vi "UHR-Fleezers Control (host) - 12.7.vi"() -> ()   [LabVIEW 2012] (continued)
        n2479 = To Double Precision Float(number=w3747) -> (double precision float=w3746:dbl[])
        n2480 = To Double Precision Float(number=w3745) -> (double precision float=w3744:dbl[])
        n2481 = Index Array(array=w3872, index=10) -> (element=w3878:waveform(dbl))
        n2482 = Index Array(array=w3872, index=11) -> (element=w3875:waveform(dbl))
        n2483 = local read "Cycles/step (MCL)"() -> (w3828:u64)
        n2484 = Index Array(array=w3872, index="Channel") -> (element=w3874:waveform(dbl))
        n2485 = Unbundle(w3780) -> ("New Image"=w3779:T2, "New Image"=w3778:T2, "New Image"=w3751:T2, "New Image"=w3752:T2, "New Image"=w3753:T2)
        n2486 = local read "Scan steps (MCL)"() -> (w3739:u64)
        n2487 = Unbundle By Name(w3878) -> ("Y"=w3830:dbl[])
        n2488 = Unbundle By Name(w3875) -> ("Y"=w3832:dbl[])
        n2489 = local read "Scan lines (y)"() -> (w3740:u64)
        n2490 = local read "N APD Samp/step"() -> (w3742:dbl)
        n2491 = Unbundle By Name(w3874) -> ("Y"=w3837:dbl[])
        n2492 = call "downsample 1D array - double.vi"("Ave N"=w3828, "Array In"=w3830) -> ("Array Out"=w3829:dbl[])  [unwired: 1 out]
        n2493 = call "downsample 1D array - double.vi"("Ave N"=w3828, "Array In"=w3832) -> ("Array Out"=w3831:dbl[])  [unwired: 1 out]
        n2494 = call "downsample 1D array - double.vi"("Ave N"=w3828, "Array In"=w3837) -> ("Array Out"=w3836:dbl[])  [unwired: 1 out]
        n2495 = Multiply(x=w3739, y=u64 2) -> (x*y=w3741:u64)
        n2496 = feedback #11(w3746) -> (w3805:dbl[])
        n2497 = Build Array (concatenate)(w3805, w3746) -> (w3804:dbl[])
        n2498 = feedback #12(w3744) -> (w3777:dbl[])
        n2499 = Build Array (concatenate)(w3777, w3744) -> (w3738:dbl[])
        n2500 = Select(t=w3746, s=w3743, f=w3804) -> (s? t:f=w3789:dbl[])
        n2501 = feedback-in #11(w3789) -> ()
        n2502 = Select(t=w3744, s=w3743, f=w3738) -> (s? t:f=w3762:dbl[])
        n2503 = feedback-in #12(w3762) -> ()
        n2504 = feedback #13(w3748) -> (w3898:dbl[])
        n2505 = Build Array (concatenate)(w3898, w3748) -> (w3880:dbl[])
        n2506 = Select(t=w3748, s=w3743, f=w3880) -> (s? t:f=w3884:dbl[])
        n2507 = feedback-in #13(w3884) -> ()
        n2508 = feedback #14(w3829) -> (w3886:dbl[])
        n2509 = Build Array (concatenate)(w3886, w3829) -> (w3877:dbl[])
        n2510 = feedback #15(w3836) -> (w3896:dbl[])
        n2511 = Build Array (concatenate)(w3896, w3836) -> (w3895:dbl[])
        n2512 = feedback #16(w3831) -> (w3888:dbl[])
        n2513 = Build Array (concatenate)(w3888, w3831) -> (w3889:dbl[])
        n2514 = Select(t=w3829, s=w3743, f=w3877) -> (s? t:f=w3833:dbl[])
        n2515 = feedback-in #14(w3833) -> ()
        n2516 = Select(t=w3836, s=w3743, f=w3895) -> (s? t:f=w3835:dbl[])
        n2517 = feedback-in #15(w3835) -> ()
        n2518 = Select(t=w3831, s=w3743, f=w3889) -> (s? t:f=w3834:dbl[])
        n2519 = feedback-in #16(w3834) -> ()
        n2520 = call "integrate 1D array interval - double.vi"("Ave N"=w3742, "Array In"=w3789) -> ("Array Out"=w3800:dbl[])  [unwired: 1 out]
        n2521 = call "integrate 1D array interval - double.vi"("Ave N"=w3742, "Array In"=w3762) -> ("Array Out"=w3773:dbl[])  [unwired: 1 out]
        n2522 = call "integrate 1D array interval - double.vi"("Ave N"=w3742, "Array In"=w3884) -> ("Array Out"=w3883:dbl[])  [unwired: 1 out]
        n2523 = Array Size(array=w3800) -> (size(s)=w3801:i32)
        n2524 = Array Size(array=w3773) -> (size(s)=w3774:i32)
        n2525 = Array Size(array=w3883) -> (size(s)=w3885:i32)
        n2526 = Multiply(x=w3740, y=w3741) -> (x*y=w3803:u64)
        n2527 = Multiply(x=w3740, y=w3741) -> (x*y=w3776:u64)
        n2528 = Multiply(x=w3740, y=w3741) -> (x*y=w3893:u64)
        n2529 = Subtract(x=w3803, y=w3801) -> (x-y=w3794:u64)
        n2530 = call-poly <vilib>:"Mean.vi"("X"=w3800) -> ("mean"=w3791:dbl)  [unwired: 1 out]
        n2531 = Subtract(x=w3776, y=w3774) -> (x-y=w3767:u64)
        n2532 = call-poly <vilib>:"Mean.vi"("X"=w3773) -> ("mean"=w3764:dbl)  [unwired: 1 out]
        n2533 = Subtract(x=w3893, y=w3885) -> (x-y=w3827:u64)
        n2534 = call-poly <vilib>:"Mean.vi"("X"=w3883) -> ("mean"=w3824:dbl)  [unwired: 1 out]
        n2535 = call-poly <vilib>:"Mean.vi"("X"=w3833) -> ("mean"=w3817:dbl)  [unwired: 1 out]
        n2536 = call-poly <vilib>:"Mean.vi"("X"=w3835) -> ("mean"=w3822:dbl)  [unwired: 1 out]
        n2537 = call-poly <vilib>:"Mean.vi"("X"=w3834) -> ("mean"=w3820:dbl)  [unwired: 1 out]
        n2538 = Initialize Array(1.0 ("element"), w3794) -> (w3790:dbl[])
        n2539 = Initialize Array(1.0 ("element"), w3767) -> (w3763:dbl[])
        n2540 = Initialize Array(1.0 ("element"), w3827) -> (w3818:dbl[])
        n2541 = Multiply(x=w3790, y=w3791) -> (x*y=w3792:dbl[])
        n2542 = Multiply(x=w3763, y=w3764) -> (x*y=w3765:dbl[])
        n2543 = Multiply(x=w3818, y=w3824) -> (x*y=w3825:dbl[])
        n2544 = Multiply(x=w3818, y=w3820) -> (x*y=w3821:dbl[])
        n2545 = Multiply(x=w3818, y=w3822) -> (x*y=w3823:dbl[])
        n2546 = Multiply(x=w3818, y=w3817) -> (x*y=w3819:dbl[])
        n2547 = Build Array (concatenate)(w3800, w3792) -> (w3802:dbl[])
        n2548 = Build Array (concatenate)(w3773, w3765) -> (w3775:dbl[])
        n2549 = Build Array (concatenate)(w3883, w3825) -> (w3892:dbl[])
        n2550 = Build Array (concatenate)(w3833, w3819) -> (w3887:dbl[])
        n2551 = Build Array (concatenate)(w3835, w3823) -> (w3891:dbl[])
        n2552 = Build Array (concatenate)(w3834, w3821) -> (w3890:dbl[])
        n2553 = Reshape Array(w3802, w3740, w3741) -> (w3798:dbl[][])
        n2554 = Reshape Array(w3775, w3740, w3741) -> (w3771:dbl[][])
        n2555 = Reshape Array(w3892, w3740, w3741) -> (w3870:dbl[][])
        n2556 = Reshape Array(w3887, w3740, w3741) -> (w3853:dbl[][])
        n2557 = Reshape Array(w3891, w3740, w3741) -> (w3845:dbl[][])
        n2558 = Reshape Array(w3890, w3740, w3741) -> (w3860:dbl[][])
        n2559 = Array Subset(array=w3798, index (col)=0 ("index"), length (col)=w3739) -> (w3797:dbl[][])  [unwired: 2 in]
        n2560 = Array Subset(array=w3798, index (col)=w3739) -> (w3795:dbl[][])  [unwired: 3 in]
        n2561 = Array Subset(array=w3771, index (col)=0 ("index"), length (col)=w3739) -> (w3770:dbl[][])  [unwired: 2 in]
        n2562 = Array Subset(array=w3771, index (col)=w3739) -> (w3768:dbl[][])  [unwired: 3 in]
        n2563 = Array Subset(array=w3860, index (col)=0 ("index"), length (col)=w3739) -> (w3865:dbl[][])  [unwired: 2 in]
        n2564 = Array Subset(array=w3860, index (col)=w3739) -> (w3863:dbl[][])  [unwired: 3 in]
        n2565 = Array Subset(array=w3870, index (col)=0 ("index"), length (col)=w3739) -> (w3869:dbl[][])  [unwired: 2 in]
        n2566 = Array Subset(array=w3870, index (col)=w3739) -> (w3867:dbl[][])  [unwired: 3 in]
        n2567 = Array Subset(array=w3845, index (col)=0 ("index"), length (col)=w3739) -> (w3851:dbl[][])  [unwired: 2 in]
        n2568 = Array Subset(array=w3845, index (col)=w3739) -> (w3849:dbl[][])  [unwired: 3 in]
        n2569 = Array Subset(array=w3853, index (col)=0 ("index"), length (col)=w3739) -> (w3858:dbl[][])  [unwired: 2 in]
        n2570 = Array Subset(array=w3853, index (col)=w3739) -> (w3856:dbl[][])  [unwired: 3 in]
        n2571 = for {
          tunnel: w3797 -> [w3902] mode=indexing
          tunnel: [w3901] -> w3796 mode=indexing
          workers-P: _ -> [_]
          n2572 = Reverse 1D Array(array=w3902) -> (reversed array=w3901:dbl[])
        }
        n2573 = for {
          tunnel: w3770 -> [w3900] mode=indexing
          tunnel: [w3899] -> w3769 mode=indexing
          workers-P: _ -> [_]
          n2574 = Reverse 1D Array(array=w3900) -> (reversed array=w3899:dbl[])
        }
        n2575 = for {
          tunnel: w3865 -> [w3908] mode=indexing
          tunnel: [w3907] -> w3864 mode=indexing
          workers-P: _ -> [_]
          n2576 = Reverse 1D Array(array=w3908) -> (reversed array=w3907:dbl[])
        }
        n2577 = for {
          tunnel: w3869 -> [w3910] mode=indexing
          tunnel: [w3909] -> w3868 mode=indexing
          workers-P: _ -> [_]
          n2578 = Reverse 1D Array(array=w3910) -> (reversed array=w3909:dbl[])
        }
        n2579 = for {
          tunnel: w3851 -> [w3904] mode=indexing
          tunnel: [w3903] -> w3850 mode=indexing
          workers-P: _ -> [_]
          n2580 = Reverse 1D Array(array=w3904) -> (reversed array=w3903:dbl[])
        }
        n2581 = for {
          tunnel: w3858 -> [w3906] mode=indexing
          tunnel: [w3905] -> w3857 mode=indexing
          workers-P: _ -> [_]
          n2582 = Reverse 1D Array(array=w3906) -> (reversed array=w3905:dbl[])
        }
        n2583 = Index Array(array=w3870, index (row)=0) -> (element=→"Waveform Graph":dbl[])  [unwired: 1 in]
        n2584 = Add(x=w3796, y=w3795) -> (x+y=w3782:dbl[][])
        n2585 = Add(x=w3769, y=w3768) -> (x+y=w3755:dbl[][])
        n2586 = Add(x=w3864, y=w3863) -> (x+y=w3862:dbl[][])
        n2587 = Add(x=w3868, y=w3867) -> (x+y=w3842:dbl[][])
        n2588 = Add(x=w3850, y=w3849) -> (x+y=w3848:dbl[][])
        n2589 = Add(x=w3857, y=w3856) -> (x+y=w3855:dbl[][])
        n2590 = Divide(x=w3848, y=2) -> (x/y=w3846:dbl[][])
        n2591 = Divide(x=w3862, y=2) -> (x/y=w3807:dbl[][])
        n2592 = To Single Precision Float(number=w3842) -> (single precision float=w3841:sgl[][])
        n2593 = To Single Precision Float(number=w3782) -> (single precision float=w3786:sgl[][])
        n2594 = To Single Precision Float(number=w3755) -> (single precision float=w3759:sgl[][])
        n2595 = Divide(x=w3855, y=2) -> (x/y=w3809:dbl[][])
        n2596 = Transpose 2D Array(2D array=w3846) -> (transposed array=→"Data map":dbl[][])
        n2597 = To Single Precision Float(number=w3807) -> (single precision float=w3813:sgl[][])
        n2598 = To Single Precision Float(number=w3809) -> (single precision float=w3810:sgl[][])
        n2599 = call "IMAQ ArrayToImage"("Image Pixels (Float)"=w3841, "Image"=w3779) -> ("Image Out"=w3844:T2)  [unwired: 8 in, 1 out]
        n2600 = call "IMAQ ArrayToImage"("Image Pixels (Float)"=w3786, "Image"=w3778) -> ("Image Out"=w3788:T2)  [unwired: 8 in, 1 out]
        n2601 = call "IMAQ ArrayToImage"("Image Pixels (Float)"=w3759, "Image"=w3751) -> ("Image Out"=w3761:T2)  [unwired: 8 in, 1 out]
        n2602 = call "IMAQ ArrayToImage"("Image Pixels (Float)"=w3813, "Image"=w3752) -> ("Image Out"=w3815:T2)  [unwired: 8 in, 1 out]
        n2603 = call "IMAQ Symmetry"("Type of Symmetry"=w3843, "Image Src"=w3844) -> ("Image Dst Out"=w3839:T2)  [unwired: 3 in, 1 out]
        n2604 = call "IMAQ ArrayToImage"("Image Pixels (Float)"=w3810, "Image"=w3753) -> ("Image Out"=w3812:T2)  [unwired: 8 in, 1 out]
        n2605 = call "IMAQ Symmetry"("Type of Symmetry"=w3787, "Image Src"=w3788) -> ("Image Dst Out"=w3784:T2)  [unwired: 3 in, 1 out]
        n2606 = call "IMAQ Symmetry"("Type of Symmetry"=w3760, "Image Src"=w3761) -> ("Image Dst Out"=w3757:T2)  [unwired: 3 in, 1 out]
        n2607 = call "IMAQ Symmetry"("Type of Symmetry"=w3814, "Image Src"=w3815) -> ("Image Dst Out"=→"Detection Laser X":T2)  [unwired: 3 in, 1 out]
        n2608 = call "IMAQ Symmetry"("Type of Symmetry"=w3811, "Image Src"=w3812) -> ("Image Dst Out"=→"Detection Laser Y":T2)  [unwired: 3 in, 1 out]
        n2609 = call "IMAQ Set Simple Calibration"("Calibration Axis Info"=T36 {"Origin Pixel"={"X"=0.0, "Y"=0.0}, "Angle Relative to Horizontal (deg)"=0.0, "Axis Reference"=0}, "Grid Descriptor"=T37 {"X Step"=0.3, "Y Step"=0.3, "Unit"=enum."Undefined"}, "Image"=w3839) -> ("Calibrated Image"=→"APD 1":T2)  [unwired: 7 in, 1 out]
        n2610 = call "IMAQ Set Simple Calibration"("Calibration Axis Info"=T36 {"Origin Pixel"={"X"=0.0, "Y"=0.0}, "Angle Relative to Horizontal (deg)"=0.0, "Axis Reference"=0}, "Grid Descriptor"=T37 {"X Step"=0.3, "Y Step"=0.3, "Unit"=enum."Undefined"}, "Image"=w3784) -> ("Calibrated Image"=→"APD 2":T2)  [unwired: 7 in, 1 out]
        n2611 = call "IMAQ Set Simple Calibration"("Calibration Axis Info"=T36 {"Origin Pixel"={"X"=0.0, "Y"=0.0}, "Angle Relative to Horizontal (deg)"=0.0, "Axis Reference"=0}, "Grid Descriptor"=T37 {"X Step"=0.3, "Y Step"=0.3, "Unit"=enum."Undefined"}, "Image"=w3757) -> ("Calibrated Image"=→"APD 3":T2)  [unwired: 7 in, 1 out]
      }
    }
    n2612 = case "For computing FFTs for display" shown="True" "Compute FFT" {
      tunnel: w3256 -> [_ w4382]
      frame False {
      }
      frame True {
        n2613 = Build Array("FFT 1 Choice 1", "FFT 1 Choice 2", "FFT 2 Choice 1", "FFT 2 Choice 2") -> (w4375:u16[])
        n2614 = Array Size(array=w4382) -> (size(s)=w4381:i32)
        n2615 = feedback-in #17(w4375) -> ()
        n2616 = feedback #17(u16[] [100, 100, 100, 100]) -> (w4376:u16[])
        n2617 = feedback-in #18("# Spectra to Ave.") -> ()
        n2618 = feedback #18("# Spectra to Ave.") -> (w4373:dbl)
        n2619 = Not Equal?(x="# Spectra to Ave.", y=w4373) -> (x != y?=w4372:bool)
        n2620 = Not Equal?(x=w4375, y=w4376) -> (x != y?=w4374:bool)
        n2621 = feedback #19(1.0) -> (w4359:dbl)
        n2622 = Compound Arithmetic op=OR("Reset FFT", w4374, w4372) -> (w4357:bool)
        n2623 = Select(t=1.0, s=w4357, f=w4359) -> (s? t:f=w4361:dbl)
        n2624 = Greater?(x=w4361, y="# Spectra to Ave.") -> (0:w4380:bool)
        n2625 = Increment(x=w4361) -> (x+1=w4360:dbl)
        n2626 = feedback-in #19(w4360) -> ()
        n2627 = local read "DMA Update Period (s)"() -> (w4355:dbl)
        n2628 = Multiply(x="# Spectra to Ave.", y=w4355) -> (x*y=→"Ave. Time (s)":dbl)
        n2629 = Build Array(cluster{"f0":dbl, "df":dbl, "magnitude":dbl[]} {"f0"=0.0, "df"=0.0, "magnitude"=[]} ("PSD")) -> (w4364:cluster{"f0":dbl, "df":dbl, "magnitude":dbl[]}[])
        n2630 = Build Array(w4364, w4364, w4364, w4364) -> (w4366:T46)
        n2631 = feedback #20(w4366) -> (w4371:T46)
        n2632 = for {
          N: 4 -> [_]
          tunnel: w4375 -> [w4404] mode=indexing
          tunnel: w4382 -> [w4405]
          tunnel: w4381 -> [w4407]
          tunnel: w4357 -> [w4400]
          tunnel: w4380 -> [w4399]
          tunnel: "# Spectra to Ave." -> [w4398]
          tunnel: [w4397] -> w4370 mode=indexing
          tunnel: w4371 -> [w4402] mode=indexing
          tunnel: [w4401] -> w4358 mode=indexing
          tunnel: w4361 -> [w4396]
          n2633 = Less?(x=w4404, y=w4407) -> (x < y?=w4406:bool)
          n2634 = Index Array(array=w4405, index=w4404) -> (element=w4403:waveform(dbl))
          n2635 = case shown="True" w4406 {
            tunnel: w4403 -> [_ w4424]
            tunnel: w4402 -> [w4409 w4422]
            tunnel: [w4409 w4410] -> w4401
            tunnel: w4400 -> [_ w4421]
            tunnel: w4399 -> [_ w4414]
            tunnel: w4398 -> [_ w4413]
            tunnel: [cluster{"f0":dbl, "df":dbl, "magnitude":dbl[]} {"f0"=0.0, "df"=0.0, "magnitude"=[]} ("PSD") w4415] -> w4397
            tunnel: w4396 -> [_ w4412]
            frame False {
            }
            frame True {
              n2636 = call <vilib>:"Std Deviation and Variance.vi"("X"=w4424) -> ("mean"=w4425:dbl)  [unwired: 1 in, 2 out]
              n2637 = Subtract(x=w4424, y=w4425) -> (x-y=w4423:waveform(dbl))
              n2638 = xnode "Spectral Measurements"("Signals"=w4423) -> ("PSD"=w4417:cluster{"f0":dbl, "df":dbl, "magnitude":dbl[]})  [unwired: 1 in, 1 out]
              n2639 = case shown="False" w4421 {
                tunnel: w4422 -> [w4434 _]
                tunnel: [w4430 w4439] -> w4410
                tunnel: w4417 -> [w4433 w4440]
                tunnel: w4414 -> [w4432 _]
                frame False {
                  n2640 = Build Array (concatenate)(w4434, w4433) -> (w4431:cluster{"f0":dbl, "df":dbl, "magnitude":dbl[]}[])
                  n2641 = case shown="True" w4432 {
                    tunnel: w4431 -> [w4435 w4438]
                    tunnel: [w4435 w4436] -> w4430
                    frame False {
                    }
                    frame True {
                      n2642 = Delete From Array(array=w4438, index=0) -> (array with subset deleted=w4436:cluster{"f0":dbl, "df":dbl, "magnitude":dbl[]}[])  [unwired: 1 in, 1 out]
                    }
                  }
                }
                frame True {
                  n2643 = Build Array(w4440) -> (w4439:cluster{"f0":dbl, "df":dbl, "magnitude":dbl[]}[])
                }
              }
              n2644 = for {
                tunnel: w4410 -> [w4429] mode=indexing
                tunnel: [w4428] -> w4420 mode=indexing
                workers-P: _ -> [_]
                n2645 = Unbundle By Name(w4429) -> ("magnitude"=w4428:dbl[])
              }
              n2646 = Transpose 2D Array(2D array=w4420) -> (transposed array=w4419:dbl[][])
              n2647 = for {
                tunnel: w4419 -> [w4427] mode=indexing
                tunnel: [w4426] -> w4418 mode=indexing
                workers-P: _ -> [_]
                n2648 = Add Array Elements(numeric array=w4427) -> (sum=w4426:dbl)
              }
              n2649 = Select(t=w4413, s=w4414, f=w4412) -> (s? t:f=w4411:dbl)
              n2650 = Divide(x=w4418, y=w4411) -> (x/y=w4416:dbl[])
              n2651 = Bundle By Name(cluster=w4417, "magnitude"=w4416) -> (w4415:cluster{"f0":dbl, "df":dbl, "magnitude":dbl[]})
            }
          }
        }
        n2652 = case shown="True" w4357 {
          tunnel: w4358 -> [w4389 w4395]
          tunnel: [w4389 w4390] -> w4356
          frame False {
          }
          frame True {
            n2653 = Array Subset(array=w4395, index (row)=0 ("index"), length (row)=4 ("length"), index (col)=0 ("index"), length (col)=1 ("length")) -> (w4390:T46)
          }
        }
        n2654 = feedback-in #20(w4356) -> ()
        n2655 = Split 1D Array(array=w4370, index=2) -> (first subarray=→"FFT 1":cluster{"f0":dbl, "df":dbl, "magnitude":dbl[]}[], second subarray=→"FFT 2":cluster{"f0":dbl, "df":dbl, "magnitude":dbl[]}[])
      }
    }
    n2656 = Index Array(array=w3254, index=4) -> (element=w3310:waveform(dbl))
    n2657 = Index Array(array=w3254, index=7) -> (element=w3307:waveform(dbl))
    n2658 = Divide(x="T1 offset_x (mV)", y=1000.0) -> (x/y=w3311:dbl)
    n2659 = feedback-in #21("Calibration") -> ()
    n2660 = feedback #21(u16 1 ("Calibration")) -> (w3329:u16)
    n2661 = Divide(x="T2 offset_x (mV)", y=1000.0) -> (x/y=w3309:dbl)
    n2662 = case shown="2" "Calibration" {
      tunnel: "T1 alpha_x (nm/V)" -> [_ w3703 w3724]
      tunnel: "T1 kappa_x (pN/nm)" -> [_ _ w3714]
      tunnel: "T2 alpha_x (nm/V)" -> [_ w3702 w3722]
      tunnel: "T2 kappa_x (pN/nm)" -> [_ _ w3715]
      tunnel: w3310 -> [w3685 w3700 w3720]
      tunnel: w3307 -> [w3684 w3698 w3718]
      tunnel: [w3685 w3697 w3717] -> w3338
      tunnel: [w3684 w3696 w3716] -> w3337
      tunnel: ["T1 X (V)" ("Label.Text") "T1 X (nm)" ("Label.Text") "T1 X (pN)" ("Label.Text")] -> w3326
      tunnel: ["T2 X (V)" ("Label.Text") "T2 X (nm)" ("Label.Text") "T2 X (pN)" ("Label.Text")] -> w3325
      tunnel: ["Position (V)" ("Label.Text") "Position (nm)" ("Label.Text") "Force (pN)" ("Label.Text")] -> w3327
      tunnel: w3309 -> [_ w3688 w3707]
      tunnel: w3311 -> [_ w3691 w3709]
      tunnel: ["Mean (V)" ("Label.Text") "Mean (nm)" ("Label.Text") "Mean (pN)" ("Label.Text")] -> w3322
      tunnel: ["Difference (V)" ("Label.Text") "Difference (nm)" ("Label.Text") "Difference (pN)" ("Label.Text")] -> w3262
      frame 0, Default {
      }
      frame 1 {
        n2663 = Unbundle By Name(w3700) -> ("Y"=w3704:dbl[])
        n2664 = Unbundle By Name(w3698) -> ("Y"=w3689:dbl[])
        n2665 = Subtract(x=w3704, y=w3691) -> (x-y=w3692:dbl[])
        n2666 = Subtract(x=w3689, y=w3688) -> (x-y=w3690:dbl[])
        n2667 = Multiply(x=w3690, y=w3702) -> (x*y=w3699:dbl[])
        n2668 = Multiply(x=w3703, y=w3692) -> (x*y=w3701:dbl[])
        n2669 = Bundle By Name(cluster=w3698, "Y"=w3699) -> (w3696:waveform(dbl))
        n2670 = Bundle By Name(cluster=w3700, "Y"=w3701) -> (w3697:waveform(dbl))
      }
      frame 2 {
        n2671 = Unbundle By Name(w3720) -> ("Y"=w3725:dbl[])
        n2672 = Unbundle By Name(w3718) -> ("Y"=w3723:dbl[])
        n2673 = Subtract(x=w3723, y=w3707) -> (x-y=w3708:dbl[])
        n2674 = Subtract(x=w3725, y=w3709) -> (x-y=w3710:dbl[])
        n2675 = Compound Arithmetic op=MULTIPLY(w3708, w3722, w3715) -> (w3719:dbl[])
        n2676 = Compound Arithmetic op=MULTIPLY(w3714, w3724, w3710) -> (w3721:dbl[])
        n2677 = Bundle By Name(cluster=w3718, "Y"=w3719) -> (w3716:waveform(dbl))
        n2678 = Bundle By Name(cluster=w3720, "Y"=w3721) -> (w3717:waveform(dbl))
      }
    }
    n2679 = case shown="True" "Read Lateness and Rel Phase" {
      tunnel: w3128 -> [w3640 w3673]
      tunnel: w3127 -> [w3641 w3672]
      tunnel: [w3640 w3645] -> w3304
      tunnel: [w3641 w3644] -> w3303
      frame False {
      }
      frame True {
        n2680 = xnode "Read/Write Control"("FPGA VI Reference In"=w3673, "error in"=w3672) -> ("FPGA VI Reference Out"=w3647:T20, "error out"=w3646:errorcluster, "GI Relative phase"=→"GI relative phase":i16, "Relative phase"=→"Relative phase (AI1)":i16, "AI Late Counter"=→"Late Counter (AI1)":u8, "GI Late Counter"=→"GI Late Counter":u8, "MCL Late Counter"=→"MCL Late Counter":u8, "MCL Relative Phase"=→"Relative Phase (MCL)":i16, "APD Acq Relative Phase"=→"APD Acq Relative Phase":i16, "APD 1 Gate Relative Phase"=→"APD 1 Gate Relative Phase":i16, "APD 2 Gate Relative Phase"=→"APD 2 Gate Relative Phase":i16, "APD Acq Late Counter"=→"APD Acq Late Counter":u8, "APD 1 Gate Late Counter"=→"APD 1 Gate Late Counter":u8, "APD 2 Gate Late Counter"=→"APD 2 Gate Late Counter":u8, "Green FB Relative Phase"=→"Relative phase (Green FB)":i16, "GI Relative phase 2"=→"GI relative phase 2":i16, "GI Late Counter 2"=→"GI Late Counter 2":u8, "Trap Pos FIFO Timeout"=→"Trap Pos FIFO Timeout":u16, "Trap AI FIFO Timeout"=→"Trap AI FIFO Timeout":u16, "RI Late Counter"=→"RI Late Counter":u8, "RI Relative phase"=→"RI relative phase":i16, "Green Late Counter"=→"Green AI Late Counter":u8, "BI Late Counter (AO)"=→"Late Counter (BI AO)":u8, "Blue Late Counter (D)"=→"Late Counter (BI DO)":u8, "BI Relative phase (AO)"=→"Relative phase (BI AO)":i16, "BI Relative phase (D)"=→"Relative phase (BI DO)":i16)
        n2681 = xnode "Read/Write Control"("FPGA VI Reference In"=w3647, "error in"=w3646) -> ("FPGA VI Reference Out"=w3645:T20, "error out"=w3644:errorcluster, "APD 3 Gate Late Counter"=→"APD 3 Gate Late Counter":u8, "APD 3 Gate Relative Phase"=→"APD 3 Gate Relative Phase":i16)
      }
    }
    n2682 = Not Equal?(x=w3329, y="Calibration") -> (x != y?=w3288:bool)
    n2683 = case shown="True" w3288 {
      tunnel: w3327 -> [_ w3678]
      tunnel: w3326 -> [_ w3677]
      tunnel: w3325 -> [_ w3676]
      tunnel: w3322 -> [_ w3675]
      tunnel: w3262 -> [_ w3674]
      frame False {
      }
      frame True {
        n2684 = property on="Force" class="WFChart (strict)"("YScale.NameLbl.Text"=w3678) -> ()  [unwired: 2 in, 2 out]
        n2685 = property on="T2 X" class="DigNum (strict)"("Caption.Text"=w3676) -> ()  [unwired: 2 in, 2 out]
        n2686 = property on="T1 X" class="DigNum (strict)"("Caption.Text"=w3677) -> ()  [unwired: 2 in, 2 out]
        n2687 = property on="Mean" class="DigNum (strict)"("Caption.Text"=w3675) -> ()  [unwired: 2 in, 2 out]
        n2688 = property on="Difference" class="DigNum (strict)"("Caption.Text"=w3674) -> ()  [unwired: 2 in, 2 out]
      }
    }
    n2689 = Unbundle By Name(w3310) -> ("Y"=w3313:dbl[])
    n2690 = Unbundle By Name(w3307) -> ("Y"=w3316:dbl[])
    n2691 = Subtract(x=w3313, y=w3311) -> (x-y=w3314:dbl[])
    n2692 = Subtract(x=w3316, y=w3309) -> (x-y=w3315:dbl[])
    n2693 = Multiply(x=w3315, y="T2 alpha_x (nm/V)") -> (x*y=w3110:dbl[])
    n2694 = Multiply(x="T1 alpha_x (nm/V)", y=w3314) -> (x*y=w3111:dbl[])
    n2695 = Not(x="Trap Trig. Fl.") -> (.not. x?=w3147:bool)
    n2696 = Multiply(x=w3337, y=-1.0) -> (x*y=w3318:waveform(dbl))
    n2697 = Subtract(x=w3111, y=w3110) -> (x-y=w3306:dbl[])
    n2698 = Unbundle By Name(w3337) -> ("Y"=w3278:dbl[])
    n2699 = Unbundle By Name(w3338) -> ("Y"=w3112:dbl[])
    n2700 = Negate(x=w3306) -> (-x=w3108:dbl[])
    n2701 = Build Array(w3338, w3318) -> (→"Force":waveform(dbl)[])
    n2702 = Subtract(x=w3108, y="Offset (nm)") -> (x-y=w3276:dbl[])
    n2703 = call-poly <vilib>:"Mean.vi"("X"=w3278) -> ("mean"=w3114:dbl)  [unwired: 1 out]
    "T2 X" <- w3114
    n2704 = Negate(x=w3278) -> (-x=w3279:dbl[])
    n2705 = call-poly <vilib>:"Mean.vi"("X"=w3112) -> ("mean"=w3115:dbl)  [unwired: 1 out]
    "T1 X" <- w3115
    n2706 = Negate(x=w3114) -> (-x=w3113:dbl)
    n2707 = Bundle By Name(cluster=w3310, "Y"=w3276) -> (w3253:waveform(dbl))
    "Bead Separation" <- w3253
    n2708 = Add(x=w3112, y=w3279) -> (x+y=w3280:dbl[])
    n2709 = Add(x=w3115, y=w3113) -> (x+y=w3324:dbl)
    n2710 = Subtract(x=w3115, y=w3113) -> (x-y=→"Difference":dbl)
    n2711 = Divide(x=w3280, y=2.0) -> (x/y=→"Vec Mean of T1 T2":dbl[])
    n2712 = Divide(x=w3324, y=2.0) -> (x/y=w3282:dbl)
    "Mean" <- w3282
    n2713 = feedback-in #22("Trap Trig. Fl.") -> ()
    n2714 = feedback #22("Trap Trig. Fl.") -> (w3145:bool)
    n2715 = And(x=w3147, y=w3145) -> (x .and. y?=w3146:bool)
    n2716 = case "If have just turned off triggering" shown="True" w3146 {
      tunnel: w3128 -> [_ w3475]
      tunnel: w3127 -> [_ w3474]
      frame False {
      }
      frame True {
        w3473 = FALSE ("FPGA Trap Trig")
        n2717 = xnode "Read/Write Control"("FPGA VI Reference In"=w3475, "error in"=w3474, "FPGA Trap Trig"=w3473) -> ("FPGA VI Reference Out"=w3472:T20, "error out"=w3471:errorcluster)
        n2718 = xnode "Read/Write Control"("FPGA VI Reference In"=w3472, "error in"=w3471, "TTrig?"=w3473) -> ()  [unwired: 2 out]
        n2719 = local write "Initializing"(FALSE ("Initializing")) -> ()
        n2720 = local write "Triggered"(FALSE ("Triggered")) -> ()
        n2721 = local write "Waiting"(FALSE ("Waiting")) -> ()
      }
    }
    n2722 = Not(x=w3145) -> (.not. x?=w3158:bool)
    n2723 = And(x="Trap Trig. Fl.", y=w3158) -> (x .and. y?=w3155:bool)
    n2724 = local read "Tether"() -> (w3283:bool)
    n2725 = Or(x=w3155, y="Reinitialize") -> (x .or. y?=w3141:bool)
    n2726 = feedback #23(w3151) -> (w3156:string)
    n2727 = Select(t=w3151, s=w3155, f=w3156) -> (s? t:f=w3150:string)
    n2728 = Select(t=w3151, s="Reinitialize", f=w3150) -> (s? t:f=w3149:string)
    n2729 = feedback #24(0) -> (w3153:i32)
    n2730 = feedback #25(w3276) -> (w3275:dbl[])
    n2731 = Build Array (concatenate)(w3276, w3275) -> (w3109:dbl[])
    n2732 = case "For determining if there is a tether still" shown="True" w3283 {
      tunnel: w3282 -> [_ w3599]
      frame False {
      }
      frame True {
        n2733 = Greater?(x="Lost Tether Alarm Threshold (pN)", y=w3599) -> (0:w3597:bool)
        n2734 = case shown="True" w3597 {
          frame False {
          }
          frame True {
            w3600 = FALSE ("Value (Signaling)")
            n2735 = flat-sequence {
              frame #0 {
                # "stop only if saving"
                n2736 = local read "Saving..."() -> (w3612:bool)
                n2737 = And(x=w3612, y="TA Cancel Save?") -> (x .and. y?=w3611:bool)
                n2738 = local write "Stop Saving"(w3611) -> ()
              }
              frame #1 {
                n2739 = case shown="True" "TA Green Off?" {
                  frame False {
                  }
                  frame True {
                    w3615 = FALSE ("Fl. Triggered...")
                    n2740 = local write "Fl. Triggered..."(w3615) -> ()
                    n2741 = property on="Green Laser ON" class="Bool (strict)"("Val(Sgnl)"=w3615) -> ()  [unwired: 2 in, 2 out]
                  }
                }
              }
            }
            n2742 = local read "Time tether formed"() -> (w3606:timestamp)
            n2743 = Get Date/Time In Seconds() -> (seconds since 1Jan1904=w3607:timestamp)
            n2744 = Subtract(x=w3607, y=w3606) -> (x-y=w3605:dbl)
            n2745 = Number To Decimal String(number=w3605) -> (decimal integer string=w3602:string)  [unwired: 1 out]
            n2746 = local read "Messages"() -> (w3609:string)
            n2747 = call <vilib>:"Beep.vi"() -> ()  [unwired: 3 in, 9 out]
            n2748 = Concatenate Strings("Lost tether (" ("Message to add"), w3602, " s)." ("string")) -> (w3604:string)
            n2749 = local write "Tether"(FALSE ("Tether")) -> ()
            n2750 = call "Update messages.vi"("Message to add"=w3604, "Old message string"=w3609) -> ("New message string"=w3608:string)
            n2751 = local write "Messages"(w3608) -> ()
            n2752 = property on="Fl. Triggered..." class="Bool (strict)"("Val(Sgnl)"=w3600) -> ()  [unwired: 2 in, 2 out]
            n2753 = local write "Dip for Protein"(w3600) -> ()
            n2754 = property on="Trap Pos. FB ON" class="Bool (strict)"("Val(Sgnl)"=w3600) -> ()  [unwired: 2 in, 2 out]
            n2755 = property on="Trap Trig. Fl." class="Bool (strict)"("Val(Sgnl)"=w3600) -> ()  [unwired: 2 in, 2 out]
          }
        }
      }
    }
    n2756 = case "For triggering actions based on the trap position (e.g., turning the excitation laser on if trap under feedback moves so far)" shown="True" "Trap Trig. Fl." {
      tunnel: w3136 -> [_ w3488]
      tunnel: w3149 -> [_ w3487]
      tunnel: ["" ("t") w3486] -> w3157
      tunnel: w3141 -> [_ w3485]
      tunnel: [0 ("t") w3484] -> w3154
      tunnel: w3153 -> [_ w3483]
      tunnel: w3128 -> [_ w3482]
      tunnel: w3127 -> [_ w3481]
      frame False {
      }
      frame True {
        n2757 = case shown="\"Wait for trigger\"" w3487 {
          tunnel: w3488 -> [w3505 _ _ w3553]
          tunnel: [w3502 w3534 "" ("t") w3556] -> w3486
          tunnel: w3485 -> [_ _ _ w3544]
          tunnel: [w3501 w3531 0 ("t") w3545] -> w3484
          tunnel: w3483 -> [_ w3533 _ w3551]
          tunnel: w3482 -> [w3490 w3528 _ w3547]
          tunnel: w3481 -> [w3489 w3527 _ w3546]
          frame "Wait for trigger" {
            n2758 = local read "Trap Trig. (FPGA)"() -> (w3493:bool)
            n2759 = Subtract(x=w3505, y="Mean T1 Position\nto compare (nm)") -> (x-y=w3498:dbl[])
            n2760 = call <vilib>:"Std Deviation and Variance.vi"("X"=w3498) -> ("mean"=→"mean":dbl, "standard deviation"=→"standard\ndeviation":dbl)  [unwired: 1 in, 1 out]
            n2761 = Array Max & Min(array=w3498) -> (max value=→"max value":dbl, min value=→"min value":dbl)  [unwired: 2 out]
            n2762 = Greater?(x=w3498, y="Threshold (nm)") -> (0:w3508:bool[])
            n2763 = case shown="True" w3493 {
              tunnel: w3490 -> [_ w3514]
              tunnel: w3489 -> [_ w3513]
              tunnel: [FALSE ("TTrig?") w3512] -> w3496
              frame False {
              }
              frame True {
                n2764 = xnode "Read/Write Control"("FPGA VI Reference In"=w3514, "error in"=w3513) -> ("TTrig?"=w3512:bool)  [unwired: 2 out]
              }
            }
            n2765 = Or Array Elements(Boolean array=w3508) -> (logical OR=w3495:bool)
            n2766 = Select(t=w3496, s=w3493, f=w3495) -> (s? t:f=w3494:bool)
            n2767 = Not(x=w3493) -> (.not. x?=w3492:bool)
            n2768 = And(x=w3494, y=w3492) -> (x .and. y?=w3491:bool)
            n2769 = Select(t="Triggered", s=w3494, f="Wait for trigger") -> (s? t:f=w3502:string)
            n2770 = case shown="True" w3494 {
              tunnel: [0 0] -> w3501
              tunnel: w3490 -> [_ w3519]
              tunnel: w3489 -> [_ w3518]
              frame False {
                "Waiting" <- TRUE ("Waiting")
              }
              frame True {
                n2771 = xnode "Read/Write Control"("FPGA VI Reference In"=w3519, "error in"=w3518, "TTrig?"=FALSE) -> ()  [unwired: 2 out]
                n2772 = local read "Messages"() -> (w3522:string)
                n2773 = call <vilib>:"Beep.vi"() -> ()  [unwired: 12 in]
                n2774 = call "Update messages.vi"("Message to add"="Unwinding trigger.", "Old message string"=w3522) -> ("New message string"=w3523:string)
                n2775 = local write "Messages"(w3523) -> ()
                n2776 = local write "Waiting"(FALSE ("Waiting")) -> ()
                "Triggered" <- TRUE ("Triggered")
              }
            }
            n2777 = case "Only need to turn on laser if host triggered" shown="True" w3491 {
              frame False {
              }
              frame True {
                n2778 = property on="Green Laser ON" class="Bool (strict)"("Val(Sgnl)"=TRUE ("Value (Signaling)")) -> ()  [unwired: 2 in, 2 out]
              }
            }
          }
          frame "Triggered" {
            n2779 = local read "Trap Trig. (FPGA)"() -> (w3530:bool)
            n2780 = Increment(x=w3533) -> (x+1=w3531:i32)
            n2781 = Greater Or Equal?(x=w3531, y="Fl. ON time (n)") -> (x >= y?=w3529:bool)
            n2782 = Select(t="Wait for trigger", s=w3529, f="Triggered" ("t")) -> (s? t:f=w3534:string)
            n2783 = And(x=w3529, y=w3530) -> (x .and. y?=w3526:bool)
            n2784 = case shown="True" w3526 {
              tunnel: w3528 -> [_ w3538]
              tunnel: w3527 -> [_ w3537]
              frame False {
              }
              frame True {
                n2785 = xnode "Read/Write Control"("FPGA VI Reference In"=w3538, "error in"=w3537, "FPGA Trap Trig"=TRUE) -> ()  [unwired: 2 out]
              }
            }
            n2786 = case shown="True" w3529 {
              frame False {
              }
              frame True {
                w3540 = FALSE ("Value (Signaling)")
                n2787 = local write "Triggered"(w3540) -> ()
                n2788 = local write "Waiting"(TRUE ("Waiting")) -> ()
                n2789 = property on="Green Laser ON" class="Bool (strict)"("Val(Sgnl)"=w3540) -> ()  [unwired: 2 in, 2 out]
              }
            }
          }
          frame "Do nothing" {
          }
          frame "Initialize", Default {
            n2790 = Increment(x=w3551) -> (x+1=w3555:i32)
            n2791 = Select(t=1, s=w3544, f=w3555) -> (s? t:f=w3545:i32)
            n2792 = feedback #26(w3553) -> (w3559:dbl[])
            n2793 = Build Array (concatenate)(w3553, w3559) -> (w3552:dbl[])
            n2794 = Greater Or Equal?(x=w3545, y="Wait to get offset (n)") -> (x >= y?=w3548:bool)
            n2795 = Select(t=w3553, s=w3544, f=w3552) -> (s? t:f=w3554:dbl[])
            n2796 = feedback-in #26(w3554) -> ()
            n2797 = call-poly <vilib>:"Mean.vi"("X"=w3554) -> ("mean"=w3549:dbl)  [unwired: 1 out]
            n2798 = local write "Mean T1 Position\nto compare (nm)"(w3549) -> ()
            n2799 = case shown="True" w3544 {
              tunnel: w3547 -> [_ w3565]
              tunnel: w3546 -> [_ w3564]
              frame False {
              }
              frame True {
                w3561 = FALSE ("FPGA Trap Trig")
                n2800 = xnode "Read/Write Control"("FPGA VI Reference In"=w3565, "error in"=w3564, "FPGA Trap Trig"=w3561) -> ("FPGA VI Reference Out"=w3563:T20, "error out"=w3562:errorcluster)
                n2801 = xnode "Read/Write Control"("FPGA VI Reference In"=w3563, "error in"=w3562, "TTrig?"=w3561) -> ()  [unwired: 2 out]
              }
            }
            n2802 = Select(t="Wait for trigger", s=w3548, f="Initialize") -> (s? t:f=w3556:string)
            n2803 = case shown="True" w3548 {
              tunnel: w3549 -> [_ w3568]
              tunnel: w3547 -> [_ w3577]
              tunnel: w3546 -> [_ w3576]
              frame False {
                n2804 = local write "Waiting"(FALSE ("Waiting")) -> ()
                "Initializing" <- TRUE ("Initializing")
              }
              frame True {
                n2805 = local read "Threshold (nm)"() -> (w3580:dbl)
                n2806 = local read "AOM X Cal (nm/MHz)"() -> (w3579:dbl)
                n2807 = Add(x=w3568, y=w3580) -> (x+y=w3581:dbl)
                n2808 = Divide(x=w3581, y=w3579) -> (x/y=w3578:dbl)
                n2809 = call "IR AOM freq to word.vi"("Frequency In (MHz)"=w3578) -> ("Frequency Word Out (double)"=w3575:dbl)
                n2810 = local write "Initializing"(FALSE ("Initializing")) -> ()
                n2811 = local write "Waiting"(TRUE ("Waiting")) -> ()
                n2812 = To Quad Integer(1:w3575) -> (0:w3574:i64)
                n2813 = xnode "Read/Write Control"("FPGA VI Reference In"=w3577, "error in"=w3576, "FPGA TTrig Thresh"=w3574) -> ("FPGA VI Reference Out"=w3571:T20, "error out"=w3570:errorcluster)
                n2814 = xnode "Read/Write Control"("FPGA VI Reference In"=w3571, "error in"=w3570, "FPGA Trap Trig"=TRUE) -> ()  [unwired: 2 out]
              }
            }
          }
        }
      }
    }
    n2815 = feedback-in #23(w3157) -> ()
    n2816 = feedback-in #24(w3154) -> ()
    n2817 = Split 1D Array(array=w3109, index=w3171) -> (first subarray=w3272:dbl[])  [unwired: 1 out]
    n2818 = feedback-in #25(w3272) -> ()
    n2819 = call-poly <vilib>:"Mean.vi"("X"=w3272) -> ("mean"=w3271:dbl)  [unwired: 1 out]
    "Bead Mean (nm)" <- w3271
    n2820 = Subtract(x=w3272, y=w3271) -> (x-y=w3270:dbl[])
    n2821 = Square(x=w3270) -> (x^2=w3269:dbl[])
    n2822 = call-poly <vilib>:"Mean.vi"("X"=w3269) -> ("mean"=w3268:dbl)  [unwired: 1 out]
    n2823 = Square Root(x=w3268) -> (sqrt(x)=w3267:dbl)
    n2824 = Multiply(x=10.0, y=w3267) -> (x*y=→"RMS (Ang)":dbl)
    n2825 = xnode ("Read/Write Control")("FPGA VI Reference In"=w3304, "error in"=w3303) -> ("FPGA VI Reference Out"=w3139:T20, "error out"=w3138:errorcluster, "AI2 Y Sum Set 1"=w3402:i16, "AI2 Y Sum Set 2"=w3401:i16, "AI1 X Set 1"=w3203:fxp<+/-,16,1>, "AI1 X Set 2"=w3202:fxp<+/-,16,1>, "Trap Pos FB Int Signal"=→"Trap Pos FB Int Signal":fxp<+/-,24,9>, "Trap Pos FB Int-Norm Signal"=→"Trap Pos FB Int-Norm Signal":fxp<+/-,16,1>, "Trap Pos FB Action"=w3196:i64, "Scanning"=→"AOD Scanning":bool, "Scan I"=→"AOD Scan I":u64, "Scanning MCL"=w3404:bool, "Scan I (MCL)"=→"MCL Scan I":u64, "Green FB Sum"=w3341:i16, "Trap Pos FB Action"=w3126:i64, "TTrig Fin Thresh"=w3122:i64, "Red FB Intensity"=w3103:i16, "Blue Intensity"=w3098:i16)
    "MCL Scanning" <- w3404
    "Trap Pos FB Action" <- w3196
    n2826 = Divide(x=w3103, y=3276.7) -> (x/y=w3102:dbl)
    "Red laser intensity (V)" <- w3102
    n2827 = Divide(x=w3098, y=3276.7) -> (x/y=w3097:dbl)
    "Blue laser intensity (V)" <- w3097
    n2828 = Divide(x=w3341, y=3276.7) -> (x/y=w3101:dbl)
    "Green laser intensity (V)" <- w3101
    n2829 = local read "FB Trig Integrate"() -> (w3120:u32)
    n2830 = Divide(x=w3126, y=w3120) -> (x/y=w3119:dbl)
    "TTrig Sig (Int)" <- w3119
    n2831 = Bundle(w3101, w3102, w3097) -> (→"Fluorescence laser intensities plot":cluster{dbl, dbl, dbl})  [unwired: 1 in]
    n2832 = Divide(x=w3122, y=w3120) -> (x/y=w3117:dbl)
    "TTrig Fin Thresh (Int)" <- w3117
    n2833 = local read "AOM X Cal (nm/MHz)"() -> (w3125:dbl)
    n2834 = local read "AI2 (V)"() -> (w3403:cluster{"Set 1":dbl, "Set 2":dbl})
    n2835 = Bundle By Name(cluster=w3403, "Set 1"=w3402, "Set 2"=w3401) -> (w3399:cluster{"Set 1":dbl, "Set 2":dbl})
    n2836 = Divide(x=w3196, y=327.67) -> (x/y=→"Action (%)":dbl)
    n2837 = local read "Trap X (AI1)"() -> (w3216:T10)
    n2838 = call "IR AOM word double to freq.vi"("Frequency Word In (double)"=w3117) -> ("Frequency Out (MHz)"=w3116:dbl)
    n2839 = call "IR AOM word double to freq.vi"("Frequency Word In (double)"=w3119) -> ("Frequency Out (MHz)"=w3118:dbl)
    n2840 = Divide(x=w3399, y=3276.7) -> (x/y=w3398:cluster{"Set 1":dbl, "Set 2":dbl})
    n2841 = Multiply(x=w3118, y=w3125) -> (x*y=w3124:dbl)
    "TTrig Sig (nm)" <- w3124
    n2842 = Multiply(x=w3116, y=w3125) -> (x*y=w3123:dbl)
    "TTrig Fin Thresh (nm)" <- w3123
    n2843 = local write "AI2 (V)"(w3398) -> ()
    n2844 = Bundle(cluster=w3216, "Trap 1"=w3203, "Trap 2"=w3202) -> (→"Trap X (AI1)":T10)
    n2845 = Bundle(w3124, w3123) -> (→"TTrig":cluster{dbl, dbl})  [unwired: 1 in]
    n2846 = flat-sequence "To save data" {
      tunnel: [w4488] -> w3422
      tunnel: [w4489] -> w3421
      tunnel: w3372 -> [w4482]
      tunnel: w3144 -> [w4486]
      tunnel: ["Save Calibration"] -> w3395
      tunnel: w3392 -> [w4485]
      tunnel: [w4478] -> w3391
      tunnel: [w4475] -> w3390
      tunnel: [w4472] -> w3389
      tunnel: w3371 -> [w4474]
      tunnel: w3286 -> [w4468]
      tunnel: [w4468] -> w3285
      tunnel: ["Start Saving"] -> w3255
      tunnel: [w4462] -> w3184
      tunnel: [w4461] -> w3183
      tunnel: w3422 -> [w4736]
      tunnel: w3421 -> [w4735]
      tunnel: w3185 -> [w4734]
      tunnel: w3395 -> [w4733]
      tunnel: w3391 -> [w4731]
      tunnel: w3390 -> [w4730]
      tunnel: w3389 -> [w4729]
      tunnel: w3264 -> [w4728]
      tunnel: w3296 -> [w4727]
      tunnel: w3285 -> [w4726]
      tunnel: w3255 -> [w4725]
      tunnel: w3253 -> [w4724]
      tunnel: w3081 -> [w4723]
      tunnel: w3184 -> [w4722]
      tunnel: w3183 -> [w4721]
      tunnel: w3182 -> [w4720]
      tunnel: w3105 -> [w4719]
      frame #0 {
        n2847 = Or(x="Save N Sets", y="Start Saving") -> (x .or. y?=w4469:bool)
        n2848 = To Double Precision Float(number=w4485) -> (double precision float=w4479:dbl)
        n2849 = Build Array(w4469, "Save Calibration", w4482, w4474) -> (w4484:bool[])
        n2850 = Compound Arithmetic op=OR("Save Calibration", w4482, w4469, w4474) -> (w4487:bool)
        n2851 = Boolean Array To Number(Boolean array=w4484) -> (number=w4481:u32)
        n2852 = feedback #27(FALSE ("Save APD Data\nwith Trap Data")) -> (w4463:bool)
        n2853 = feedback #28(refnum<k0> refnum) -> (w4490:refnum<file>)
        n2854 = feedback #29(refnum<k0> refnum) -> (w4465:refnum<file>)
        n2855 = feedback #30(FALSE ("Save APD Data\nwith Trap Data")) -> (w4473:bool)
        n2856 = feedback #31(refnum<k0> refnum) -> (w4476:refnum<file>)
        n2857 = feedback #32(0) -> (w4492:i32)
        n2858 = feedback #33() -> (w4480:u32)  [unwired: 1 out]
        n2859 = case shown="True" w4487 {
          tunnel: [w4499 1] -> w4488
          tunnel: w4492 -> [w4501 _]
          tunnel: [w4500 w4532] -> w4489
          tunnel: w4490 -> [w4500 _]
          tunnel: w4486 -> [_ w4550]
          tunnel: w4479 -> [_ w4548]
          tunnel: w4481 -> [_ w4551]
          tunnel: [w4498 w4531] -> w4478
          tunnel: w4480 -> [w4498 _]
          tunnel: [w4497 w4529] -> w4475
          tunnel: w4476 -> [w4497 _]
          tunnel: [w4496 w4528] -> w4472
          tunnel: w4473 -> [w4496 _]
          tunnel: "Start Saving" -> [_ w4526]
          tunnel: w4468 -> [_ w4525]
          tunnel: [w4495 w4517] -> w4461
          tunnel: w4465 -> [w4495 _]
          tunnel: [w4494 w4516] -> w4462
          tunnel: w4463 -> [w4494 _]
          frame False {
            n2860 = Increment(x=w4501) -> (x+1=w4499:i32)
          }
          frame True {
            w4522 = FALSE ("Start Saving")
            w4527 = 9.0  # File Version
            w4534 = FALSE ("prepend array or string size? (T)")
            w4533 = T28."big-endian, network order" ("byte order (0:big-endian, network order)")
            n2861 = local read "BD 1 Frequency 1 (MHz)"() -> (w4547:dbl)
            n2862 = local read "BD 2 Frequency 1 (MHz)"() -> (w4546:dbl)
            n2863 = local read "BD 1 Frequency 2 (MHz)"() -> (w4545:dbl)
            n2864 = local read "BD 2 Frequency 2 (MHz)"() -> (w4544:dbl)
            n2865 = local read "BD 1 Frequency 3 (MHz)"() -> (w4543:dbl)
            n2866 = local read "BD 2 Frequency 3 (MHz)"() -> (w4542:dbl)
            n2867 = Array Size(array=w4525) -> (size(s)=w4524:i32)
            n2868 = To Double Precision Float(number=w4524) -> (double precision float=w4523:dbl)
            n2869 = local write "Save Calibration"(w4522) -> ()
            n2870 = local write "Start Saving"(w4522) -> ()
            n2871 = Build Array("Save APD Data\nwith Trap Data", "Save Trap Pos. Data") -> (w4519:bool[])
            n2872 = Boolean Array To Number(Boolean array=w4519) -> (number=w4518:u32)
            n2873 = Build Array(w4547, w4546, w4545, w4544, w4543, w4542) -> (w4541:dbl[])
            n2874 = case shown="1, Default" w4551 {
              tunnel: w4550 -> [w4623 w4643 w4659 w4697]
              tunnel: w4523 -> [w4628 w4650 w4679 w4716]
              tunnel: w4548 -> [w4627 w4649 w4678 w4715]
              tunnel: [w4624 w4645 w4670 w4707] -> w4539
              tunnel: [w4615 "Cal sets to save" w4660 w4698] -> w4531
              tunnel: w4541 -> [w4625 w4646 w4672 w4709]
              tunnel: "Save APD Data\nwith Trap Data" -> [w4622 _ w4656 w4695]
              tunnel: [w4622 w4637 w4656 w4695] -> w4528
              tunnel: w4527 -> [w4618 w4638 w4654 w4693]
              tunnel: w4526 -> [w4617 _ _ _]
              tunnel: [w4608 w4637 w4653 w4683] -> w4516
              tunnel: "Save Trap Pos. Data" -> [w4608 _ w4653 w4683]
              tunnel: w4518 -> [w4607 _ w4652 w4682]
              frame 1, Default {
                # "timeseries"
                n2875 = case shown="True" "Profile" {
                  tunnel: [w4631 w4635] -> w4612
                  tunnel: [w4631 w4634] -> w4611
                  tunnel: [w4631 w4633] -> w4610
                  tunnel: [w4631 w4632] -> w4609
                  frame False {
                    w4631 = 0.0 ("f")
                  }
                  frame True {
                    n2876 = local read "Current Position"() -> (w4636:cluster{dbl, dbl, dbl})
                    n2877 = local read "Y change (mm)"() -> (w4632:dbl)
                    n2878 = Unbundle(w4636) -> (w4635:dbl, w4634:dbl, w4633:dbl)
                  }
                }
                n2879 = local read "Save ave N"() -> (w4630:dbl)
                n2880 = Multiply(x=w4630, y=w4623) -> (x*y=w4629:dbl)
                n2881 = To Double Precision Float(number=w4607) -> (double precision float=w4621:dbl)
                n2882 = Build Array(w4618, w4623, w4629, w4628, w4627, 0.0 ("f")) -> (w4626:dbl[])
                n2883 = Build Array(w4621, w4612, w4611, w4610, w4609) -> (w4619:dbl[])
                n2884 = Select(t=u32 4000000000, s=w4617, f="N sets to save") -> (s? t:f=w4615:u32)
                n2885 = Build Array (concatenate)(w4626, w4625, w4619) -> (w4624:dbl[])
              }
              frame 2 {
                w4640 = 0.0 ("f")
                w4637 = FALSE ("Save APD Data\nwith Trap Data")
                # "calibration"
                n2886 = Boolean To (0,1)(Boolean=w4637) -> (0, 1=w4642:i16)
                n2887 = To Double Precision Float(number=w4642) -> (double precision float=w4641:dbl)
                n2888 = Build Array(w4641, w4640, w4640, w4640, w4640) -> (w4639:dbl[])
                n2889 = Build Array(w4638, w4643, w4643, w4650, w4649, 1.0 ("t")) -> (w4647:dbl[])
                n2890 = Build Array (concatenate)(w4647, w4646, w4639) -> (w4645:dbl[])
                "Calibrating Trap..." <- TRUE ("Calibrating...")
              }
              frame 4 {
                w4657 = 0.0 ("f")
                # "scan dir (x/y = 0/1)"
                # "cycles/step"
                # "n scans (f/b)"
                # "steps"
                # "freq. range"
                # "AOD raster scan"
                n2891 = local read "Number of F/B Scans (AOD)"() -> (w4664:u16)
                n2892 = local read "Cycles/step (AOD)"() -> (w4666:u64)
                n2893 = local read "Scan Range (MHz)"() -> (w4669:dbl)
                n2894 = local read "Scan steps (AOD)"() -> (w4668:u64)
                n2895 = local read "Scan BD"() -> (w4676:bool)
                n2896 = local read "Save ave N"() -> (w4681:dbl)
                n2897 = Boolean To (0,1)(Boolean=w4676) -> (0, 1=w4675:i16)
                n2898 = To Double Precision Float(number=w4664) -> (double precision float=w4663:dbl)
                n2899 = To Double Precision Float(number=w4668) -> (double precision float=w4667:dbl)
                n2900 = To Double Precision Float(number=w4666) -> (double precision float=w4665:dbl)
                n2901 = To Double Precision Float(number=w4675) -> (double precision float=w4674:dbl)
                n2902 = Multiply(x=w4681, y=w4659) -> (x*y=w4680:dbl)
                n2903 = To Double Precision Float(number=w4652) -> (double precision float=w4658:dbl)
                n2904 = Build Array(w4658, w4657, w4657, w4657, w4657) -> (w4655:dbl[])
                n2905 = local read "N sets should be saved"() -> (w4661:dbl)
                n2906 = Build Array(w4674, w4669, w4667, w4665, w4663) -> (w4671:dbl[])
                n2907 = Build Array(w4654, w4659, w4680, w4679, w4678, 2.0 ("t")) -> (w4673:dbl[])
                n2908 = Round Toward +Infinity(x=w4661) -> (ceil(x): smallest int >= x=w4662:dbl)
                n2909 = Build Array (concatenate)(w4673, w4672, w4655, w4671) -> (w4670:dbl[])
                n2910 = To Unsigned Long Integer(number=w4662) -> (unsigned 32bit integer=w4660:u32)
              }
              frame 8 {
                w4690 = 0.0 ("f")
                # "MCL raster scan"
                n2911 = local read "Number of scans (MCL)"() -> (w4685:u64)
                n2912 = local read "Scan lines (y)"() -> (w4684:u64)
                n2913 = local read "2D or 1D Scan"() -> (w4687:bool)
                n2914 = local read "Scan Range (V)\n(of steps)"() -> (w4706:dbl)
                n2915 = local read "Fast Scan Dir"() -> (w4713:bool)
                n2916 = local read "Cycles/step (MCL)"() -> (w4703:u64)
                n2917 = local read "Scan steps (MCL)"() -> (w4705:u64)
                n2918 = Select(t=w4684, s=w4687, f=w4685) -> (s? t:f=w4686:u64)
                n2919 = Boolean To (0,1)(Boolean=w4687) -> (0, 1=w4689:i16)
                n2920 = local read "Save ave N"() -> (w4718:dbl)
                n2921 = local read "Initial X"() -> (w4692:dbl)
                n2922 = local read "Initial Y"() -> (w4691:dbl)
                n2923 = To Double Precision Float(number=w4689) -> (double precision float=w4688:dbl)
                n2924 = Boolean To (0,1)(Boolean=w4713) -> (0, 1=w4712:i16)
                n2925 = To Double Precision Float(number=w4686) -> (double precision float=w4701:dbl)
                n2926 = To Double Precision Float(number=w4705) -> (double precision float=w4704:dbl)
                n2927 = To Double Precision Float(number=w4703) -> (double precision float=w4702:dbl)
                n2928 = To Double Precision Float(number=w4712) -> (double precision float=w4711:dbl)
                n2929 = Multiply(x=w4718, y=w4697) -> (x*y=w4717:dbl)
                n2930 = To Double Precision Float(number=w4682) -> (double precision float=w4696:dbl)
                n2931 = local read "N sets should be saved (MCL)"() -> (w4699:dbl)
                n2932 = Build Array(w4696, w4688, w4690, w4690, w4690) -> (w4694:dbl[])
                n2933 = Build Array(w4711, w4706, w4704, w4702, w4701, w4692, w4691) -> (w4708:dbl[])
                n2934 = Build Array(w4693, w4697, w4717, w4716, w4715, 3.0 ("t")) -> (w4710:dbl[])
                n2935 = Round Toward +Infinity(x=w4699) -> (ceil(x): smallest int >= x=w4700:dbl)
                n2936 = Build Array (concatenate)(w4710, w4709, w4694, w4708) -> (w4707:dbl[])
                n2937 = To Unsigned Long Integer(number=w4700) -> (unsigned 32bit integer=w4698:u32)
              }
            }
            n2938 = local read "Index"() -> (w4556:dbl)
            n2939 = call "Create new save file.vi"("Insert"="", "Ext"=".dat", "Index In"=w4556) -> ("Path Out"=w4512:path, "Index Out"=w4530:dbl)
            n2940 = local write "Save file name"(w4512) -> ()
            n2941 = local write "Index"(w4530) -> ()
            n2942 = local write "Save index"(w4530) -> ()
            n2943 = Array Size(array=w4539) -> (size(s)=w4540:i32)
            n2944 = Open/Create/Replace File(file path (use dialog)=w4512, operation (0:open)=T29."create", access (0:read/write)=enum16{"read/write", "read-only", "write-only"}."write-only") -> (refnum out=w4553:refnum<file>)  [unwired: 1 in, 4 out]
            n2945 = local write "Saving..."(TRUE ("Saving...")) -> ()
            n2946 = To Double Precision Float(number=w4540) -> (double precision float=w4538:dbl)
            n2947 = String Length(string="Comment (data description)") -> (length=w4537:i32)
            n2948 = To Double Precision Float(number=w4537) -> (double precision float=w4536:dbl)
            n2949 = Deny Access(7:w4553) -> (3:w4552:refnum<file>)  [unwired: 1 in, 2 out]
            n2950 = Build Array (concatenate)(w4538, w4539, w4536) -> (w4511:dbl[])
            n2951 = case "If fluorescence data to be saved" shown="True" w4528 {
              tunnel: w4512 -> [_ w4606]